vi "Dresden R2R Sputter 03.02.2018 IY24.vi"() -> ()   [LabVIEW 2009] (continued)
                                frame #1 {
                                }
                                }
                                }
                                }
                              }
                              frame #1 {
                              }
                            }
                          }
                          frame #8 {
                            # "OPEN PC-BV"
                            n19406 = local read "Semi"() -> (w24101:bool)
                            n19407 = case shown="False" w24101 {
                              frame #0 {
                                n19408 = stacked-sequence {
                                frame #0 {
                                n19409 = local read "Semi"() -> (w24102:bool)
                                n19410 = case shown="False" w24102 {
                                frame #0 {
                                n19411 = stacked-sequence {
                                frame #0 {
                                n19412 = local read "Semi"() -> (w24103:bool)
                                n19413 = case shown="False" w24103 {
                                frame #0 {
                                n19414 = local write "Pc_bv3_auto_open"(TRUE ("Tp1_auto_start")) -> ()
                                }
                                frame #1 {
                                }
                                }
                                }
                                frame #1 {
                                n19415 = local read "Semi"() -> (w24105:bool)
                                n19416 = case shown="False" w24105 {
                                frame #0 {
                                n19417 = Wait (ms)(milliseconds to wait=u32 1000) -> ()  [unwired: 1 out]
                                }
                                frame #1 {
                                }
                                }
                                }
                                frame #2 {
                                n19418 = local read "Semi"() -> (w24107:bool)
                                n19419 = case shown="False" w24107 {
                                frame #0 {
                                n19420 = while {
                                i -> [w24113]
                                stop <- w24109 stop-if-true
                                n19421 = local read "Pc_bv_opened_ch3"() -> (w24111:bool)
                                n19422 = Greater?(x=w24113, y=120) -> (0:w24112:bool)
                                n19423 = local read "Semi"() -> (w24110:bool)
                                n19424 = Compound Arithmetic op=OR(w24110, w24111, w24112) -> (w24109:bool)
                                n19425 = Wait (ms)(milliseconds to wait=u32 500) -> ()  [unwired: 1 out]
                                }
                                }
                                frame #1 {
                                }
                                }
                                }
                                frame #3 {
                                n19426 = local read "Semi"() -> (w24115:bool)
                                n19427 = case shown="False" w24115 {
                                frame #0 {
                                n19428 = local read "Pc_bv_opened_ch3"() -> (w24116:bool)
                                n19429 = case shown="False" w24116 {
                                frame #0 {
                                n19430 = local write "Pc_bv3_auto_open"(TRUE ("Pc_bv1_auto_open")) -> ()
                                }
                                frame #1 {
                                }
                                }
                                }
                                frame #1 {
                                }
                                }
                                }
                                frame #4 {
                                n19431 = local read "Semi"() -> (w24118:bool)
                                n19432 = case shown="False" w24118 {
                                frame #0 {
                                n19433 = local read "Pc_bv_opened_ch3"() -> (w24119:bool)
                                n19434 = case shown="False" w24119 {
                                frame #0 {
                                n19435 = Wait (ms)(milliseconds to wait=u32 1000) -> ()  [unwired: 1 out]
                                }
                                frame #1 {
                                }
                                }
                                }
                                frame #1 {
                                }
                                }
                                }
                                frame #5 {
                                n19436 = local read "Semi"() -> (w24121:bool)
                                n19437 = case shown="False" w24121 {
                                frame #0 {
                                n19438 = while {
                                i -> [w24127]
                                stop <- w24123 stop-if-true
                                n19439 = local read "Pc_bv_opened_ch3"() -> (w24125:bool)
                                n19440 = Greater?(x=w24127, y=120) -> (0:w24126:bool)
                                n19441 = local read "Semi"() -> (w24124:bool)
                                n19442 = Compound Arithmetic op=OR(w24124, w24125, w24126) -> (w24123:bool)
                                n19443 = Wait (ms)(milliseconds to wait=u32 500) -> ()  [unwired: 1 out]
                                }
                                }
                                frame #1 {
                                }
                                }
                                }
                                frame #6 {
                                n19444 = local read "Semi"() -> (w24129:bool)
                                n19445 = case shown="False" w24129 {
                                frame #0 {
                                n19446 = local read "Pc_bv_opened_ch3"() -> (w24130:bool)
                                n19447 = case shown="False" w24130 {
                                frame #0 {
                                n19448 = local write "Error Message"("Start up process  cancelled\nbecause  PC-BV not opened.\nPlease check PC-BV3 connections." ("Error Message")) -> ()
                                n19449 = Wait (ms)(milliseconds to wait=u32 1000) -> ()  [unwired: 1 out]
                                }
                                frame #1 {
                                }
                                }
                                }
                                frame #1 {
                                }
                                }
                                }
                                }
                                }
                                frame #1 {
                                }
                                }
                                }
                                frame #1 {
                                n19450 = local read "Semi"() -> (w24133:bool)
                                n19451 = case shown="False" w24133 {
                                frame #0 {
                                n19452 = local write "Ch3_PV14"(TRUE ("P03")) -> ()
                                n19453 = Wait Until Next ms Multiple(millisecond multiple=u32 1000) -> ()  [unwired: 1 out]
                                }
                                frame #1 {
                                }
                                }
                                }
                                }
                              }
                              frame #1 {
                              }
                            }
                          }
                          frame #9 {
                            # "OPEN/CLOSE TRNS GV-BP2"
                            n19454 = local read "Semi"() -> (w24136:bool)
                            n19455 = case shown="False" w24136 {
                              frame #0 {
                                n19456 = stacked-sequence {
                                frame #0 {
                                n19457 = local read "Semi"() -> (w24137:bool)
                                n19458 = case shown="False" w24137 {
                                frame #0 {
                                n19459 = while {
                                i -> [w24146]
                                stop <- w24141 stop-if-true
                                n19460 = Greater?(x=w24146, y=800) -> (0:w24144:bool)
                                n19461 = case shown="True" w24144 {
                                frame #0 {
                                }
                                frame #1 {
                                n19462 = local read "Ch4pressure"() -> (w24160:dbl)
                                n19463 = Less?(x=w24160, y=1) -> (x < y?=w24159:bool)
                                n19464 = case shown="False" w24159 {
                                frame #0 {
                                n19465 = local write "Error Message"("Start up process  cancelled\nbecause \n Trns GV-BP2 not closed.\nPlease check \nTrns GV-BP2 connections." ("Error Message")) -> ()
                                }
                                frame #1 {
                                n19466 = local write "Error Message"("Start up process  cancelled\nbecause \n Trns GV-BP2 not opened.\nPlease check \nTrns GV-BP2 connections." ("Error Message")) -> ()
                                }
                                }
                                n19467 = local write "Semi"(TRUE ("Semi")) -> ()
                                }
                                }
                                n19468 = local read "Ch4pressure"() -> (w24140:dbl)
                                n19469 = Less?(x=w24140, y=1) -> (x < y?=w24138:bool)
                                n19470 = case shown="True" w24138 {
                                tunnel: [w24148 w24154] -> w24143
                                frame #0 {
                                n19471 = local read "Ch3_Trns_gv_bp2_di"() -> (w24147:bool)
                                n19472 = case shown="True" w24147 {
                                tunnel: [TRUE FALSE] -> w24148
                                frame #0 {
                                }
                                frame #1 {
                                n19473 = local write "Ch3_Trns_gv_bp2_do"(FALSE ("Ch1_Tp_bv_do")) -> ()
                                n19474 = Wait Until Next ms Multiple(millisecond multiple=u32 200) -> ()  [unwired: 1 out]
                                }
                                }
                                }
                                frame #1 {
                                n19475 = local read "Ch3_Trns_gv_bp2_di"() -> (w24153:bool)
                                n19476 = case shown="False" w24153 {
                                tunnel: [FALSE TRUE] -> w24154
                                frame #0 {
                                n19477 = local write "Ch3_Trns_gv_bp2_do"(TRUE ("Ch1_Tp_bv_do")) -> ()
                                n19478 = Wait Until Next ms Multiple(millisecond multiple=u32 200) -> ()  [unwired: 1 out]
                                }
                                frame #1 {
                                }
                                }
                                }
                                }
                                n19479 = local read "Semi"() -> (w24142:bool)
                                n19480 = Or(x=w24143, y=w24142) -> (x .or. y?=w24141:bool)
                                }
                                }
                                frame #1 {
                                }
                                }
                                }
                                frame #1 {
                                n19481 = local read "Semi"() -> (w24165:bool)
                                n19482 = case shown="False" w24165 {
                                frame #0 {
                                n19483 = local write "Ch3_PV15"(TRUE ("P03")) -> ()
                                n19484 = Wait Until Next ms Multiple(millisecond multiple=u32 1000) -> ()  [unwired: 1 out]
                                }
                                frame #1 {
                                }
                                }
                                }
                                }
                              }
                              frame #1 {
                              }
                            }
                          }
                          frame #10 {
                            # "OPEN/CLOSE TRNS GV-BP"
                            n19485 = local read "Semi"() -> (w24168:bool)
                            n19486 = case shown="False" w24168 {
                              frame #0 {
                                n19487 = stacked-sequence {
                                frame #0 {
                                n19488 = local read "Semi"() -> (w24169:bool)
                                n19489 = case shown="False" w24169 {
                                frame #0 {
                                n19490 = while {
                                i -> [w24178]
                                stop <- w24173 stop-if-true
                                n19491 = Greater?(x=w24178, y=800) -> (0:w24176:bool)
                                n19492 = case shown="True" w24176 {
                                frame #0 {
                                }
                                frame #1 {
                                n19493 = local read "Ch2_pressure"() -> (w24192:dbl)
                                n19494 = Less?(x=w24192, y=1) -> (x < y?=w24191:bool)
                                n19495 = case shown="True" w24191 {
                                frame #0 {
                                n19496 = local write "Error Message"("Start up process  cancelled\nbecause \n Trns GV-BP not closed.\nPlease check \nTrns GV-BP connections." ("Error Message")) -> ()
                                }
                                frame #1 {
                                n19497 = local write "Error Message"("Start up process  cancelled\nbecause \n Trns GV-BP not opened.\nPlease check \nTrns GV-BP connections." ("Error Message")) -> ()
                                }
                                }
                                n19498 = local write "Semi"(TRUE ("Semi")) -> ()
                                }
                                }
                                n19499 = local read "Ch2_pressure"() -> (w24172:dbl)
                                n19500 = Less?(x=w24172, y=1) -> (x < y?=w24170:bool)
                                n19501 = case shown="True" w24170 {
                                tunnel: [w24180 w24186] -> w24175
                                frame #0 {
                                n19502 = local read "Ch3_Trns_gv_bp_di"() -> (w24179:bool)
                                n19503 = case shown="True" w24179 {
                                tunnel: [TRUE FALSE] -> w24180
                                frame #0 {
                                }
                                frame #1 {
                                n19504 = local write "Ch3_Trns_gv_bp_do"(FALSE ("Ch1_Tp_bv_do")) -> ()
                                n19505 = Wait Until Next ms Multiple(millisecond multiple=u32 200) -> ()  [unwired: 1 out]
                                }
                                }
                                }
                                frame #1 {
                                n19506 = local read "Ch3_Trns_gv_bp_di"() -> (w24185:bool)
                                n19507 = case shown="False" w24185 {
                                tunnel: [FALSE TRUE] -> w24186
                                frame #0 {
                                n19508 = local write "Ch3_Trns_gv_bp_do"(TRUE ("Ch1_Tp_bv_do")) -> ()
                                n19509 = Wait Until Next ms Multiple(millisecond multiple=u32 200) -> ()  [unwired: 1 out]
                                }
                                frame #1 {
                                }
                                }
                                }
                                }
                                n19510 = local read "Semi"() -> (w24174:bool)
                                n19511 = Or(x=w24175, y=w24174) -> (x .or. y?=w24173:bool)
                                }
                                }
                                frame #1 {
                                }
                                }
                                }
                                frame #1 {
                                n19512 = local read "Semi"() -> (w24197:bool)
                                n19513 = case shown="False" w24197 {
                                frame #0 {
                                n19514 = local write "Ch3_PV16"(TRUE ("P03")) -> ()
                                n19515 = Wait Until Next ms Multiple(millisecond multiple=u32 1000) -> ()  [unwired: 1 out]
                                }
                                frame #1 {
                                }
                                }
                                }
                                }
                              }
                              frame #1 {
                              }
                            }
                          }
                          frame #11 {
                            # "CHECK CH-PRESSURE"
                            n19516 = local read "Semi"() -> (w24200:bool)
                            n19517 = case shown="False" w24200 {
                              frame #0 {
                                n19518 = stacked-sequence {
                                frame #0 {
                                n19519 = local read "Semi"() -> (w24201:bool)
                                n19520 = case shown="False" w24201 {
                                frame #0 {
                                n19521 = while {
                                i -> [w24210]
                                stop <- w24205 stop-if-true
                                n19522 = Greater?(x=w24210, y=600) -> (0:w24208:bool)
                                n19523 = case shown="True" w24208 {
                                frame #0 {
                                }
                                frame #1 {
                                n19524 = local write "Semi"(TRUE ("Semi")) -> ()
                                n19525 = local write "Error Message"("Start up process was cancelled.\nPlease check chamber \nvacuum connections." ("Error Message")) -> ()
                                }
                                }
                                n19526 = local read "Ch3_pressure"() -> (w24204:dbl)
                                n19527 = Less?(x=w24204, y=0.9) -> (x < y?=w24202:bool)
                                n19528 = case shown="False" w24202 {
                                tunnel: [FALSE TRUE] -> w24207
                                frame #0 {
                                n19529 = Wait Until Next ms Multiple(millisecond multiple=u32 500) -> ()  [unwired: 1 out]
                                }
                                frame #1 {
                                }
                                }
                                n19530 = local read "Semi"() -> (w24206:bool)
                                n19531 = Or(x=w24207, y=w24206) -> (x .or. y?=w24205:bool)
                                }
                                }
                                frame #1 {
                                }
                                }
                                }
                                frame #1 {
                                n19532 = local read "Semi"() -> (w24216:bool)
                                n19533 = case shown="False" w24216 {
                                frame #0 {
                                n19534 = local write "Ch3_PV17"(TRUE ("P03")) -> ()
                                n19535 = Wait Until Next ms Multiple(millisecond multiple=u32 1000) -> ()  [unwired: 1 out]
                                }
                                frame #1 {
                                }
                                }
                                }
                                }
                              }
                              frame #1 {
                              }
                            }
                          }
                          frame #12 {
                            # "OPEN BG-BV"
                            n19536 = local read "Semi"() -> (w24219:bool)
                            n19537 = case shown="False" w24219 {
                              frame #0 {
                                n19538 = stacked-sequence {
                                frame #0 {
                                n19539 = local read "Semi"() -> (w24220:bool)
                                n19540 = case shown="False" w24220 {
                                frame #0 {
                                n19541 = while {
                                i -> [w24227]
                                stop <- w24222 stop-if-true
                                n19542 = Greater?(x=w24227, y=50) -> (0:w24225:bool)
                                n19543 = case shown="True" w24225 {
                                frame #0 {
                                }
                                frame #1 {
                                n19544 = local write "Semi"(TRUE ("Semi")) -> ()
                                n19545 = local write "Error Message"("Start up process  cancelled\nbecause  BG-BV not opened.\nPlease check BG-BV3 connections." ("Error Message")) -> ()
                                }
                                }
                                n19546 = local read "Ch3_Bg_bv_di"() -> (w24221:bool)
                                n19547 = case shown="False" w24221 {
                                tunnel: [FALSE TRUE] -> w24224
                                frame #0 {
                                n19548 = Wait Until Next ms Multiple(millisecond multiple=u32 200) -> ()  [unwired: 1 out]
                                n19549 = local write "Ch3_Bg_bv_do"(TRUE ("Ch1_Tp_bv_do")) -> ()
                                }
                                frame #1 {
                                }
                                }
                                n19550 = local read "Semi"() -> (w24223:bool)
                                n19551 = Or(x=w24224, y=w24223) -> (x .or. y?=w24222:bool)
                                }
                                }
                                frame #1 {
                                }
                                }
                                }
                                frame #1 {
                                n19552 = local read "Semi"() -> (w24234:bool)
                                n19553 = case shown="False" w24234 {
                                frame #0 {
                                n19554 = local write "Ch3_PV18"(TRUE ("P03")) -> ()
                                n19555 = Wait Until Next ms Multiple(millisecond multiple=u32 1000) -> ()  [unwired: 1 out]
                                }
                                frame #1 {
                                }
                                }
                                }
                                }
                              }
                              frame #1 {
                              }
                            }
                          }
                          frame #13 {
                            # "CHECK CH-PRESSURE"
                            n19556 = local read "Semi"() -> (w24237:bool)
                            n19557 = case shown="False" w24237 {
                              frame #0 {
                                n19558 = stacked-sequence {
                                frame #0 {
                                n19559 = local read "Semi"() -> (w24238:bool)
                                n19560 = case shown="False" w24238 {
                                frame #0 {
                                n19561 = while {
                                i -> [w24247]
                                stop <- w24242 stop-if-true
                                n19562 = Greater?(x=w24247, y=240) -> (0:w24245:bool)
                                n19563 = case shown="True" w24245 {
                                frame #0 {
                                }
                                frame #1 {
                                n19564 = local write "Semi"(TRUE ("Semi")) -> ()
                                n19565 = local write "Error Message"("Start up process was cancelled.\nPlease check chamber \nvacuum connections." ("Error Message")) -> ()
                                }
                                }
                                n19566 = local read "Ch3_pressure"() -> (w24241:dbl)
                                n19567 = Less?(x=w24241, y=0.9) -> (x < y?=w24239:bool)
                                n19568 = case shown="True" w24239 {
                                tunnel: [FALSE TRUE] -> w24244
                                frame #0 {
                                n19569 = Wait Until Next ms Multiple(millisecond multiple=u32 500) -> ()  [unwired: 1 out]
                                }
                                frame #1 {
                                }
                                }
                                n19570 = local read "Semi"() -> (w24243:bool)
                                n19571 = Or(x=w24244, y=w24243) -> (x .or. y?=w24242:bool)
                                }
                                }
                                frame #1 {
                                }
                                }
                                }
                                frame #1 {
                                n19572 = local read "Semi"() -> (w24253:bool)
                                n19573 = case shown="False" w24253 {
                                frame #0 {
                                n19574 = local write "Ch3_PV19"(TRUE ("P03")) -> ()
                                n19575 = Wait Until Next ms Multiple(millisecond multiple=u32 1000) -> ()  [unwired: 1 out]
                                }
                                frame #1 {
                                }
                                }
                                }
                                }
                              }
                              frame #1 {
                              }
                            }
                          }
                          frame #14 {
                            # "START TP"
                            n19576 = local read "Semi"() -> (w24256:bool)
                            n19577 = case shown="False" w24256 {
                              frame #0 {
                                n19578 = stacked-sequence {
                                frame #0 {
                                n19579 = local read "Semi"() -> (w24257:bool)
                                n19580 = case shown="False" w24257 {
                                frame #0 {
                                n19581 = stacked-sequence {
                                frame #0 {
                                n19582 = local read "Semi"() -> (w24258:bool)
                                n19583 = case shown="False" w24258 {
                                frame #0 {
                                n19584 = local write "Tp3_auto_start"(TRUE ("Tp1_auto_start")) -> ()
                                }
                                frame #1 {
                                }
                                }
                                }
                                frame #1 {
                                n19585 = local read "Semi"() -> (w24260:bool)
                                n19586 = case shown="False" w24260 {
                                frame #0 {
                                n19587 = Wait (ms)(milliseconds to wait=u32 1000) -> ()  [unwired: 1 out]
                                }
                                frame #1 {
                                }
                                }
                                }
                                frame #2 {
                                n19588 = local read "Semi"() -> (w24262:bool)
                                n19589 = case shown="False" w24262 {
                                frame #0 {
                                n19590 = while {
                                i -> [w24268]
                                stop <- w24264 stop-if-true
                                n19591 = local read "TP3_working"() -> (w24266:bool)
                                n19592 = Greater?(x=w24268, y=120) -> (0:w24267:bool)
                                n19593 = local read "Semi"() -> (w24265:bool)
                                n19594 = Compound Arithmetic op=OR(w24265, w24266, w24267) -> (w24264:bool)
                                n19595 = Wait (ms)(milliseconds to wait=u32 500) -> ()  [unwired: 1 out]
                                }
                                }
                                frame #1 {
                                }
                                }
                                }
                                frame #3 {
                                n19596 = local read "Semi"() -> (w24270:bool)
                                n19597 = case shown="False" w24270 {
                                frame #0 {
                                n19598 = local read "TP3_working"() -> (w24271:bool)
                                n19599 = case shown="False" w24271 {
                                frame #0 {
                                n19600 = local write "Tp3_auto_start"(TRUE ("Pc_bv1_auto_open")) -> ()
                                }
                                frame #1 {
                                }
                                }
                                }
                                frame #1 {
                                }
                                }
                                }
                                frame #4 {
                                n19601 = local read "Semi"() -> (w24273:bool)
                                n19602 = case shown="False" w24273 {
                                frame #0 {
                                n19603 = local read "TP3_working"() -> (w24274:bool)
                                n19604 = case shown="False" w24274 {
                                frame #0 {
                                n19605 = Wait (ms)(milliseconds to wait=u32 1000) -> ()  [unwired: 1 out]
                                }
                                frame #1 {
                                }
                                }
                                }
                                frame #1 {
                                }
                                }
                                }
                                frame #5 {
                                n19606 = local read "Semi"() -> (w24276:bool)
                                n19607 = case shown="False" w24276 {
                                frame #0 {
                                n19608 = while {
                                i -> [w24282]
                                stop <- w24278 stop-if-true
                                n19609 = local read "TP3_working"() -> (w24280:bool)
                                n19610 = Greater?(x=w24282, y=120) -> (0:w24281:bool)
                                n19611 = local read "Semi"() -> (w24279:bool)
                                n19612 = Compound Arithmetic op=OR(w24279, w24280, w24281) -> (w24278:bool)
                                n19613 = Wait (ms)(milliseconds to wait=u32 500) -> ()  [unwired: 1 out]
                                }
                                }
                                frame #1 {
                                }
                                }
                                }
                                frame #6 {
                                n19614 = local read "Semi"() -> (w24284:bool)
                                n19615 = case shown="False" w24284 {
                                frame #0 {
                                n19616 = local read "TP3_working"() -> (w24285:bool)
                                n19617 = case shown="False" w24285 {
                                frame #0 {
                                n19618 = local write "Error Message"("Start up process  cancelled\nbecause  TP not started.\nPlease check TP3 connections." ("Error Message")) -> ()
                                n19619 = Wait (ms)(milliseconds to wait=u32 1000) -> ()  [unwired: 1 out]
                                }
                                frame #1 {
                                }
                                }
                                }
                                frame #1 {
                                }
                                }
                                }
                                }
                                }
                                frame #1 {
                                }
                                }
                                }
                                frame #1 {
                                n19620 = local read "Semi"() -> (w24288:bool)
                                n19621 = case shown="False" w24288 {
                                frame #0 {
                                n19622 = local write "Ch3_PV20"(TRUE ("P03")) -> ()
                                n19623 = Wait Until Next ms Multiple(millisecond multiple=u32 1000) -> ()  [unwired: 1 out]
                                }
                                frame #1 {
                                }
                                }
                                }
                                }
                              }
                              frame #1 {
                              }
                            }
                          }
                        }
                      }
                      frame #1 {
                      }
                    }
                  }
                  frame #1 {
                    # "PUMPING CH3 HIGHER THAN 0.9 TORR"
                    n19624 = local read "Semi"() -> (w24291:bool)
                    n19625 = case shown="False" w24291 {
                      frame #0 {
                        n19626 = stacked-sequence {
                          frame #0 {
                            # "STOP TP"
                            n19627 = local read "Semi"() -> (w24292:bool)
                            n19628 = case shown="False" w24292 {
                              frame #0 {
                                n19629 = stacked-sequence {
                                frame #0 {
                                n19630 = local read "Semi"() -> (w24293:bool)
                                n19631 = case shown="False" w24293 {
                                frame #0 {
                                n19632 = stacked-sequence {
                                frame #0 {
                                n19633 = local read "Semi"() -> (w24294:bool)
                                n19634 = case shown="False" w24294 {
                                frame #0 {
                                n19635 = local write "Tp3_auto_stop"(TRUE ("Tp1_auto_start")) -> ()
                                }
                                frame #1 {
                                }
                                }
                                }
                                frame #1 {
                                n19636 = local read "Semi"() -> (w24296:bool)
                                n19637 = case shown="False" w24296 {
                                frame #0 {
                                n19638 = Wait (ms)(milliseconds to wait=u32 1000) -> ()  [unwired: 1 out]
                                }
                                frame #1 {
                                }
                                }
                                }
                                frame #2 {
                                n19639 = local read "Semi"() -> (w24298:bool)
                                n19640 = case shown="False" w24298 {
                                frame #0 {
                                n19641 = while {
                                i -> [w24304]
                                stop <- w24300 stop-if-true
                                n19642 = local read "Tp3_stopped"() -> (w24302:bool)
                                n19643 = Greater?(x=w24304, y=120) -> (0:w24303:bool)
                                n19644 = local read "Semi"() -> (w24301:bool)
                                n19645 = Compound Arithmetic op=OR(w24301, w24302, w24303) -> (w24300:bool)
                                n19646 = Wait (ms)(milliseconds to wait=u32 500) -> ()  [unwired: 1 out]
                                }
                                }
                                frame #1 {
                                }
                                }
                                }
                                frame #3 {
                                n19647 = local read "Semi"() -> (w24306:bool)
                                n19648 = case shown="False" w24306 {
                                frame #0 {
                                n19649 = local read "Tp3_stopped"() -> (w24307:bool)
                                n19650 = case shown="False" w24307 {
                                frame #0 {
                                n19651 = local write "Tp3_auto_stop"(TRUE ("Pc_bv1_auto_open")) -> ()
                                }
                                frame #1 {
                                }
                                }
                                }
                                frame #1 {
                                }
                                }
                                }
                                frame #4 {
                                n19652 = local read "Semi"() -> (w24309:bool)
                                n19653 = case shown="False" w24309 {
                                frame #0 {
                                n19654 = local read "Tp3_stopped"() -> (w24310:bool)
                                n19655 = case shown="False" w24310 {
                                frame #0 {
                                n19656 = Wait (ms)(milliseconds to wait=u32 1000) -> ()  [unwired: 1 out]
                                }
                                frame #1 {
                                }
                                }
                                }
                                frame #1 {
                                }
                                }
                                }
                                frame #5 {
                                n19657 = local read "Semi"() -> (w24312:bool)
                                n19658 = case shown="False" w24312 {
                                frame #0 {
                                n19659 = while {
                                i -> [w24318]
                                stop <- w24314 stop-if-true
                                n19660 = local read "Tp3_stopped"() -> (w24316:bool)
                                n19661 = Greater?(x=w24318, y=120) -> (0:w24317:bool)
                                n19662 = local read "Semi"() -> (w24315:bool)
                                n19663 = Compound Arithmetic op=OR(w24315, w24316, w24317) -> (w24314:bool)
                                n19664 = Wait (ms)(milliseconds to wait=u32 500) -> ()  [unwired: 1 out]
                                }
                                }
                                frame #1 {
                                }
                                }
                                }
                                frame #6 {
                                n19665 = local read "Semi"() -> (w24320:bool)
                                n19666 = case shown="False" w24320 {
                                frame #0 {
                                n19667 = local read "Tp3_stopped"() -> (w24321:bool)
                                n19668 = case shown="False" w24321 {
                                frame #0 {
                                n19669 = local write "Error Message"("Start up process  cancelled\nbecause  TP not stopped.\nPlease check TP3 connections." ("Error Message")) -> ()
                                n19670 = Wait (ms)(milliseconds to wait=u32 1000) -> ()  [unwired: 1 out]
                                }
                                frame #1 {
                                }
                                }
                                }
                                frame #1 {
                                }
                                }
                                }
                                }
                                }
                                frame #1 {
                                }
                                }
                                }
                                frame #1 {
                                n19671 = local read "Semi"() -> (w24324:bool)
                                n19672 = case shown="False" w24324 {
                                frame #0 {
                                n19673 = local write "Ch3_PA6"(TRUE ("PA2")) -> ()
                                n19674 = Wait Until Next ms Multiple(millisecond multiple=u32 1000) -> ()  [unwired: 1 out]
                                }
                                frame #1 {
                                }
                                }
                                }
                                }
                              }
                              frame #1 {
                              }
                            }
                          }
                          frame #1 {
                            # "CLOSE CH-CC"
                            n19675 = local read "Semi"() -> (w24327:bool)
                            n19676 = case shown="False" w24327 {
                              frame #0 {
                                n19677 = stacked-sequence {
                                frame #0 {
                                n19678 = local read "Semi"() -> (w24328:bool)
                                n19679 = case shown="False" w24328 {
                                frame #0 {
                                n19680 = while {
                                i -> [w24335]
                                stop <- w24329 stop-if-true
                                n19681 = Greater?(x=w24335, y=50) -> (0:w24333:bool)
                                n19682 = case shown="True" w24333 {
                                frame #0 {
                                }
                                frame #1 {
                                n19683 = local write "Semi"(TRUE ("Semi")) -> ()
                                n19684 = local write "Error Message"("Start up process  cancelled\nbecause  CH-CC not closed.\nPlease check  CH3-CC connections." ("Error Message")) -> ()
                                }
                                }
                                n19685 = local read "Ch3_Cc_on_off_di"() -> (w24332:bool)
                                n19686 = case shown="True" w24332 {
                                tunnel: [TRUE FALSE] -> w24331
                                frame #0 {
                                }
                                frame #1 {
                                n19687 = Wait Until Next ms Multiple(millisecond multiple=u32 200) -> ()  [unwired: 1 out]
                                n19688 = local write "Ch3_Cc_on_off_do"(FALSE ("Ch1_Tp_bv_do")) -> ()
                                }
                                }
                                n19689 = local read "Semi"() -> (w24330:bool)
                                n19690 = Or(x=w24331, y=w24330) -> (x .or. y?=w24329:bool)
                                }
                                }
                                frame #1 {
                                }
                                }
                                }